vi "run_pharmaBotExp_v0.015.vi"(0 "data in":T12={"daq_ao 1"="Dev1/ao0", "daq_ai 1"="Dev1/ai0", "experiment day folder"=path "C:/multiBot/data/debug/testing", "Multiclamp init error"=0, "Multiclamp Handle Out"=10225184, "sampling rate (Hz)"=20000, "trial name"="t1"}, 1 "auto run?":bool=TRUE, 3 "which manipulator":T13(ring), 4 "HEK/slice options":enum16{"slice", "HEK"}(ring), 5 "error in":errorcluster, 6 "Validate after Experiment":bool, 7 "common cluster":T9, 11 "individual controls in":T8, 13 "images":T3={"slice image"="remote image 000000001461186C", "pipette template"="remote image 000000001461152C", "found pipette"=refnum, "pipette mask for cell tracker"=refnum, "cell images ref"=refnum}) -> (10 "Cell Looks Good?":bool=TRUE, 12 "ValidationOutputCluster":T5(array[cluster]), 14 "ValidationResults":waveform(dbl)[][](array[waveform]), 15 "ValidationPos1":T6(array[ring]), 16 "Exp. Terminated":bool, 17 "ValidationPos2":T6(array[ring]), 18 "ValidationWaveform":waveform(dbl)[](array[waveform]), 19 "error out":errorcluster)   [LabVIEW 2015] (continued)
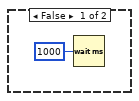
[diagram p2: hidden frame]
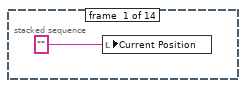
[diagram p3: hidden frame]
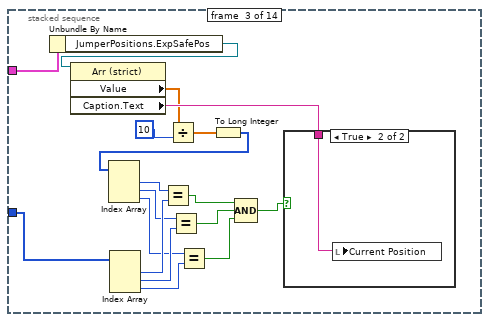
[diagram p5: hidden frame]
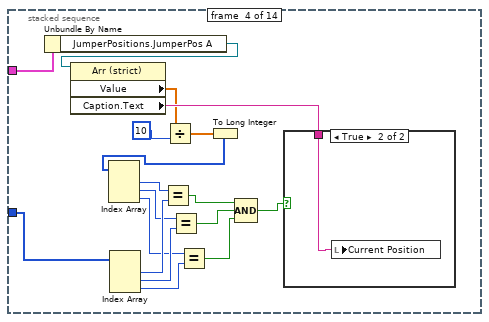
[diagram p7: hidden frame]
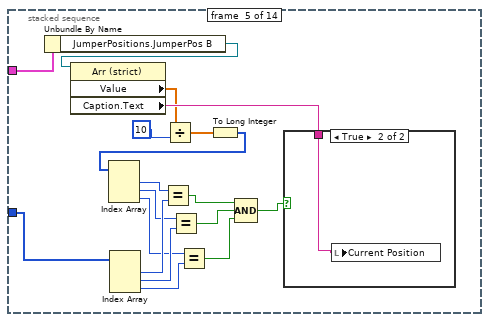
[diagram p9: hidden frame]
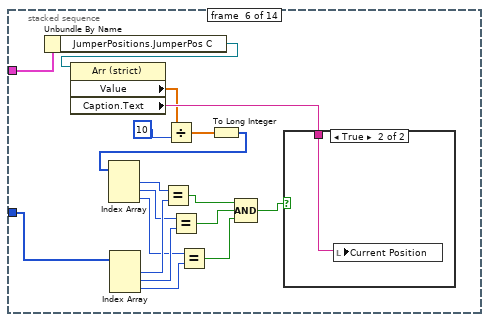
[diagram p11: hidden frame]
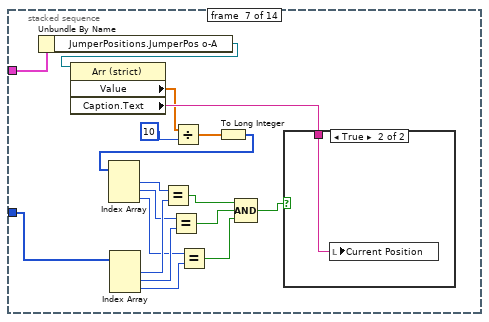
[diagram p13: hidden frame]
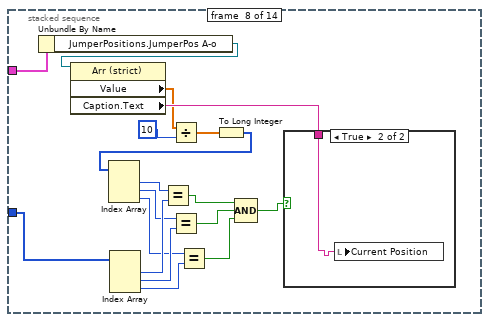
[diagram p15: hidden frame]
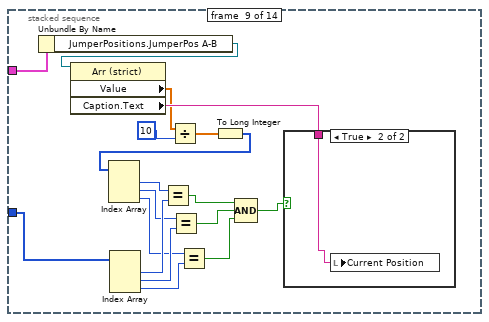
[diagram p17: hidden frame]
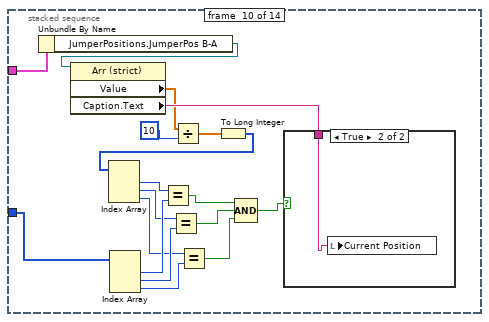
[diagram p19: hidden frame]
            n2141 = control-ref of="PhaseC Experiment Option"() -> (w2881:refnum<vi>)
            n2142 = control-ref of="PhaseE Experiment Option"() -> (w2873:refnum<vi>)
            n2143 = property class="CmbBox"(reference=w2892, "Visible"=TRUE) -> ()  [unwired: 1 in, 2 out]
            n2144 = property class="CmbBox"(reference=w2890, "Visible"=TRUE) -> ()  [unwired: 1 in, 2 out]
            n2145 = property class="CmbBox"(reference=w2872, "Visible"=TRUE) -> ()  [unwired: 1 in, 2 out]
            n2146 = property class="CmbBox"(reference=w2880, "Visible"=TRUE) -> ()  [unwired: 1 in, 2 out]
            n2147 = property class="CmbBox"(reference=w2881, "Visible"=TRUE) -> ()  [unwired: 1 in, 2 out]
            n2148 = property class="CmbBox"(reference=w2873, "Visible"=TRUE) -> ()  [unwired: 1 in, 2 out]
            n2149 = control-ref of="Experiment Selection B"() -> (w2887:refnum<vi>)
            n2150 = control-ref of="Experiment Selection F"() -> (w2869:refnum<vi>)
            n2151 = control-ref of="Experiment Selection D"() -> (w2877:refnum<vi>)
            n2152 = control-ref of="Experiment Selection A"() -> (w2885:refnum<vi>)
            n2153 = control-ref of="Experiment Selection C"() -> (w2884:refnum<vi>)
            n2154 = control-ref of="Experiment Selection E"() -> (w2876:refnum<vi>)
            n2155 = property class="TabCtl (strict)"(reference=w2887, "Visible"=TRUE) -> ()  [unwired: 1 in, 2 out]
            n2156 = property class="TabCtl (strict)"(reference=w2885, "Visible"=TRUE) -> ()  [unwired: 1 in, 2 out]
            n2157 = property class="TabCtl (strict)"(reference=w2869, "Visible"=TRUE) -> ()  [unwired: 1 in, 2 out]
            n2158 = property class="TabCtl (strict)"(reference=w2877, "Visible"=TRUE) -> ()  [unwired: 1 in, 2 out]
            n2159 = property class="TabCtl (strict)"(reference=w2884, "Visible"=TRUE) -> ()  [unwired: 1 in, 2 out]
            n2160 = property class="TabCtl (strict)"(reference=w2876, "Visible"=TRUE) -> ()  [unwired: 1 in, 2 out]
            n2161 = control-ref of="PhaseH Experiment Option"() -> (w2847:refnum<vi>)
            n2162 = control-ref of="PhaseL Experiment Option"() -> (w2865:refnum<vi>)
            n2163 = control-ref of="PhaseG Experiment Option"() -> (w2845:refnum<vi>)
            n2164 = control-ref of="PhaseJ Experiment Option"() -> (w2857:refnum<vi>)
            n2165 = control-ref of="PhaseI Experiment Option"() -> (w2856:refnum<vi>)
            n2166 = control-ref of="PhaseK Experiment Option"() -> (w2864:refnum<vi>)
            n2167 = property class="CmbBox"(reference=w2845, "Visible"=TRUE) -> ()  [unwired: 1 in, 2 out]
            n2168 = property class="CmbBox"(reference=w2847, "Visible"=TRUE) -> ()  [unwired: 1 in, 2 out]
            n2169 = property class="CmbBox"(reference=w2865, "Visible"=FALSE) -> ()  [unwired: 1 in, 2 out]
            n2170 = property class="CmbBox"(reference=w2857, "Visible"=TRUE) -> ()  [unwired: 1 in, 2 out]
            n2171 = property class="CmbBox"(reference=w2856, "Visible"=TRUE) -> ()  [unwired: 1 in, 2 out]
            n2172 = property class="CmbBox"(reference=w2864, "Visible"=FALSE) -> ()  [unwired: 1 in, 2 out]
            n2173 = control-ref of="Experiment Selection H"() -> (w2850:refnum<vi>)
            n2174 = control-ref of="Experiment Selection L"() -> (w2868:refnum<vi>)
            n2175 = control-ref of="Experiment Selection J"() -> (w2860:refnum<vi>)
            n2176 = control-ref of="Experiment Selection G"() -> (w2852:refnum<vi>)
            n2177 = control-ref of="Experiment Selection I"() -> (w2853:refnum<vi>)
            n2178 = control-ref of="Experiment Selection K"() -> (w2861:refnum<vi>)
            n2179 = property class="TabCtl (strict)"(reference=w2850, "Visible"=TRUE) -> ()  [unwired: 1 in, 2 out]
            n2180 = property class="TabCtl (strict)"(reference=w2852, "Visible"=TRUE) -> ()  [unwired: 1 in, 2 out]
            n2181 = property class="TabCtl (strict)"(reference=w2868, "Visible"=FALSE) -> ()  [unwired: 1 in, 2 out]
            n2182 = property class="TabCtl (strict)"(reference=w2860, "Visible"=TRUE) -> ()  [unwired: 1 in, 2 out]
            n2183 = property class="TabCtl (strict)"(reference=w2853, "Visible"=TRUE) -> ()  [unwired: 1 in, 2 out]
            n2184 = property class="TabCtl (strict)"(reference=w2861, "Visible"=FALSE) -> ()  [unwired: 1 in, 2 out]
          }
          frame 11 {
            n2185 = control-ref of="PhaseB Experiment Option"() -> (w2938:refnum<vi>)
            n2186 = control-ref of="PhaseF Experiment Option"() -> (w2920:refnum<vi>)
            n2187 = control-ref of="PhaseA Experiment Option"() -> (w2940:refnum<vi>)
            n2188 = control-ref of="PhaseD Experiment Option"() -> (w2928:refnum<vi>)
            n2189 = control-ref of="PhaseC Experiment Option"() -> (w2929:refnum<vi>)
            n2190 = control-ref of="PhaseE Experiment Option"() -> (w2921:refnum<vi>)
            n2191 = property class="CmbBox"(reference=w2940, "Visible"=TRUE) -> ()  [unwired: 1 in, 2 out]
            n2192 = property class="CmbBox"(reference=w2938, "Visible"=TRUE) -> ()  [unwired: 1 in, 2 out]
            n2193 = property class="CmbBox"(reference=w2920, "Visible"=TRUE) -> ()  [unwired: 1 in, 2 out]
            n2194 = property class="CmbBox"(reference=w2928, "Visible"=TRUE) -> ()  [unwired: 1 in, 2 out]
            n2195 = property class="CmbBox"(reference=w2929, "Visible"=TRUE) -> ()  [unwired: 1 in, 2 out]
            n2196 = property class="CmbBox"(reference=w2921, "Visible"=TRUE) -> ()  [unwired: 1 in, 2 out]
            n2197 = control-ref of="Experiment Selection B"() -> (w2935:refnum<vi>)
            n2198 = control-ref of="Experiment Selection F"() -> (w2917:refnum<vi>)
            n2199 = control-ref of="Experiment Selection D"() -> (w2925:refnum<vi>)
            n2200 = control-ref of="Experiment Selection A"() -> (w2933:refnum<vi>)
            n2201 = control-ref of="Experiment Selection C"() -> (w2932:refnum<vi>)
            n2202 = control-ref of="Experiment Selection E"() -> (w2924:refnum<vi>)
            n2203 = property class="TabCtl (strict)"(reference=w2935, "Visible"=TRUE) -> ()  [unwired: 1 in, 2 out]
            n2204 = property class="TabCtl (strict)"(reference=w2933, "Visible"=TRUE) -> ()  [unwired: 1 in, 2 out]
            n2205 = property class="TabCtl (strict)"(reference=w2917, "Visible"=TRUE) -> ()  [unwired: 1 in, 2 out]
            n2206 = property class="TabCtl (strict)"(reference=w2925, "Visible"=TRUE) -> ()  [unwired: 1 in, 2 out]
            n2207 = property class="TabCtl (strict)"(reference=w2932, "Visible"=TRUE) -> ()  [unwired: 1 in, 2 out]
            n2208 = property class="TabCtl (strict)"(reference=w2924, "Visible"=TRUE) -> ()  [unwired: 1 in, 2 out]
            n2209 = control-ref of="PhaseH Experiment Option"() -> (w2895:refnum<vi>)
            n2210 = control-ref of="PhaseL Experiment Option"() -> (w2913:refnum<vi>)
            n2211 = control-ref of="PhaseG Experiment Option"() -> (w2893:refnum<vi>)
            n2212 = control-ref of="PhaseJ Experiment Option"() -> (w2905:refnum<vi>)
            n2213 = control-ref of="PhaseI Experiment Option"() -> (w2904:refnum<vi>)
            n2214 = control-ref of="PhaseK Experiment Option"() -> (w2912:refnum<vi>)
            n2215 = property class="CmbBox"(reference=w2893, "Visible"=TRUE) -> ()  [unwired: 1 in, 2 out]
            n2216 = property class="CmbBox"(reference=w2895, "Visible"=TRUE) -> ()  [unwired: 1 in, 2 out]
            n2217 = property class="CmbBox"(reference=w2913, "Visible"=FALSE) -> ()  [unwired: 1 in, 2 out]
            n2218 = property class="CmbBox"(reference=w2905, "Visible"=TRUE) -> ()  [unwired: 1 in, 2 out]
            n2219 = property class="CmbBox"(reference=w2904, "Visible"=TRUE) -> ()  [unwired: 1 in, 2 out]
            n2220 = property class="CmbBox"(reference=w2912, "Visible"=TRUE) -> ()  [unwired: 1 in, 2 out]
            n2221 = control-ref of="Experiment Selection H"() -> (w2898:refnum<vi>)
            n2222 = control-ref of="Experiment Selection L"() -> (w2916:refnum<vi>)
            n2223 = control-ref of="Experiment Selection J"() -> (w2908:refnum<vi>)
            n2224 = control-ref of="Experiment Selection G"() -> (w2900:refnum<vi>)
            n2225 = control-ref of="Experiment Selection I"() -> (w2901:refnum<vi>)
            n2226 = control-ref of="Experiment Selection K"() -> (w2909:refnum<vi>)
            n2227 = property class="TabCtl (strict)"(reference=w2898, "Visible"=TRUE) -> ()  [unwired: 1 in, 2 out]
            n2228 = property class="TabCtl (strict)"(reference=w2900, "Visible"=TRUE) -> ()  [unwired: 1 in, 2 out]
            n2229 = property class="TabCtl (strict)"(reference=w2916, "Visible"=FALSE) -> ()  [unwired: 1 in, 2 out]
            n2230 = property class="TabCtl (strict)"(reference=w2908, "Visible"=TRUE) -> ()  [unwired: 1 in, 2 out]
            n2231 = property class="TabCtl (strict)"(reference=w2901, "Visible"=TRUE) -> ()  [unwired: 1 in, 2 out]
            n2232 = property class="TabCtl (strict)"(reference=w2909, "Visible"=TRUE) -> ()  [unwired: 1 in, 2 out]
          }
          frame 12 {
            n2233 = control-ref of="PhaseB Experiment Option"() -> (w2986:refnum<vi>)
            n2234 = control-ref of="PhaseF Experiment Option"() -> (w2968:refnum<vi>)
            n2235 = control-ref of="PhaseA Experiment Option"() -> (w2988:refnum<vi>)
            n2236 = control-ref of="PhaseD Experiment Option"() -> (w2976:refnum<vi>)
            n2237 = control-ref of="PhaseC Experiment Option"() -> (w2977:refnum<vi>)
            n2238 = control-ref of="PhaseE Experiment Option"() -> (w2969:refnum<vi>)
            n2239 = property class="CmbBox"(reference=w2988, "Visible"=TRUE) -> ()  [unwired: 1 in, 2 out]
            n2240 = property class="CmbBox"(reference=w2986, "Visible"=TRUE) -> ()  [unwired: 1 in, 2 out]
            n2241 = property class="CmbBox"(reference=w2968, "Visible"=TRUE) -> ()  [unwired: 1 in, 2 out]
            n2242 = property class="CmbBox"(reference=w2976, "Visible"=TRUE) -> ()  [unwired: 1 in, 2 out]
            n2243 = property class="CmbBox"(reference=w2977, "Visible"=TRUE) -> ()  [unwired: 1 in, 2 out]
            n2244 = property class="CmbBox"(reference=w2969, "Visible"=TRUE) -> ()  [unwired: 1 in, 2 out]
            n2245 = control-ref of="Experiment Selection B"() -> (w2983:refnum<vi>)
            n2246 = control-ref of="Experiment Selection F"() -> (w2965:refnum<vi>)
            n2247 = control-ref of="Experiment Selection D"() -> (w2973:refnum<vi>)
            n2248 = control-ref of="Experiment Selection A"() -> (w2981:refnum<vi>)
            n2249 = control-ref of="Experiment Selection C"() -> (w2980:refnum<vi>)
            n2250 = control-ref of="Experiment Selection E"() -> (w2972:refnum<vi>)
            n2251 = property class="TabCtl (strict)"(reference=w2983, "Visible"=TRUE) -> ()  [unwired: 1 in, 2 out]
            n2252 = property class="TabCtl (strict)"(reference=w2981, "Visible"=TRUE) -> ()  [unwired: 1 in, 2 out]
            n2253 = property class="TabCtl (strict)"(reference=w2965, "Visible"=TRUE) -> ()  [unwired: 1 in, 2 out]
            n2254 = property class="TabCtl (strict)"(reference=w2973, "Visible"=TRUE) -> ()  [unwired: 1 in, 2 out]
            n2255 = property class="TabCtl (strict)"(reference=w2980, "Visible"=TRUE) -> ()  [unwired: 1 in, 2 out]
            n2256 = property class="TabCtl (strict)"(reference=w2972, "Visible"=TRUE) -> ()  [unwired: 1 in, 2 out]
            n2257 = control-ref of="PhaseH Experiment Option"() -> (w2943:refnum<vi>)
            n2258 = control-ref of="PhaseL Experiment Option"() -> (w2961:refnum<vi>)
            n2259 = control-ref of="PhaseG Experiment Option"() -> (w2941:refnum<vi>)
            n2260 = control-ref of="PhaseJ Experiment Option"() -> (w2953:refnum<vi>)
            n2261 = control-ref of="PhaseI Experiment Option"() -> (w2952:refnum<vi>)
            n2262 = control-ref of="PhaseK Experiment Option"() -> (w2960:refnum<vi>)
            n2263 = property class="CmbBox"(reference=w2941, "Visible"=TRUE) -> ()  [unwired: 1 in, 2 out]
            n2264 = property class="CmbBox"(reference=w2943, "Visible"=TRUE) -> ()  [unwired: 1 in, 2 out]
            n2265 = property class="CmbBox"(reference=w2961, "Visible"=TRUE) -> ()  [unwired: 1 in, 2 out]
            n2266 = property class="CmbBox"(reference=w2953, "Visible"=TRUE) -> ()  [unwired: 1 in, 2 out]
            n2267 = property class="CmbBox"(reference=w2952, "Visible"=TRUE) -> ()  [unwired: 1 in, 2 out]
            n2268 = property class="CmbBox"(reference=w2960, "Visible"=TRUE) -> ()  [unwired: 1 in, 2 out]
            n2269 = control-ref of="Experiment Selection H"() -> (w2946:refnum<vi>)
            n2270 = control-ref of="Experiment Selection L"() -> (w2964:refnum<vi>)
            n2271 = control-ref of="Experiment Selection J"() -> (w2956:refnum<vi>)
            n2272 = control-ref of="Experiment Selection G"() -> (w2948:refnum<vi>)
            n2273 = control-ref of="Experiment Selection I"() -> (w2949:refnum<vi>)
            n2274 = control-ref of="Experiment Selection K"() -> (w2957:refnum<vi>)
            n2275 = property class="TabCtl (strict)"(reference=w2946, "Visible"=TRUE) -> ()  [unwired: 1 in, 2 out]
            n2276 = property class="TabCtl (strict)"(reference=w2948, "Visible"=TRUE) -> ()  [unwired: 1 in, 2 out]
            n2277 = property class="TabCtl (strict)"(reference=w2964, "Visible"=TRUE) -> ()  [unwired: 1 in, 2 out]
            n2278 = property class="TabCtl (strict)"(reference=w2956, "Visible"=TRUE) -> ()  [unwired: 1 in, 2 out]
            n2279 = property class="TabCtl (strict)"(reference=w2949, "Visible"=TRUE) -> ()  [unwired: 1 in, 2 out]
            n2280 = property class="TabCtl (strict)"(reference=w2957, "Visible"=TRUE) -> ()  [unwired: 1 in, 2 out]
          }
        }
      }
      event "Single Manip Jump A", "Single Manip Jump B", "Single Manip Jump C", "Single Manip Jump D", "Single Manip Jump E", "Single Manip Jump F", "Single Manip Jump L", "Single Manip Jump K", "Single Manip Jump J", "Single Manip Jump I", "Single Manip Jump H", "Single Manip Jump G": Value Change {
        n2281 = event-data() -> ("CtlRef"=w2992:refnum<vi>, "OldVal"=w2990:T28, "NewVal"=w2991:T28)  [unwired: 1 in, 3 out]
        n2282 = local read "Waveform Simulation sampling rate (Hz)"() -> (w2989:i32)
        n2283 = call "calc_singleManipJumpWaveform_v0.02.vi"("New input cluster"=w2991, "Old input cluster"=w2990, "simulate Wave freq"=w2989) -> ("output cluster"=w2993:T28)  [unwired: 11 in, 1 out]
        n2284 = property class="Clust (strict)"(reference=w2992, "Value"=w2993) -> ()  [unwired: 1 in, 2 out]
      }
      event "Multi Manip Jump A", "Multi Manip Jump B", "Multi Manip Jump C", "Multi Manip Jump D", "Multi Manip Jump E", "Multi Manip Jump F", "Multi Manip Jump L", "Multi Manip Jump K", "Multi Manip Jump J", "Multi Manip Jump I", "Multi Manip Jump H", "Multi Manip Jump G": Value Change {
        n2285 = event-data() -> ("CtlRef"=w2997:refnum<vi>, "OldVal"=w2995:T30, "NewVal"=w2996:T30)  [unwired: 1 in, 3 out]
        n2286 = local read "Waveform Simulation sampling rate (Hz)"() -> (w2994:i32)
        n2287 = call "calc_multiManipJumpWaveform_v0.02.vi"("New input cluster"=w2996, "Old input cluster"=w2995, "Numeric"=w2994) -> ("output cluster"=w2998:T30)  [unwired: 11 in, 1 out]
        n2288 = property class="Clust (strict)"(reference=w2997, "Value"=w2998) -> ()  [unwired: 1 in, 2 out]
      }
      event "Paired Pulse A", "Paired Pulse B", "Paired Pulse C", "Paired Pulse D", "Paired Pulse E", "Paired Pulse F", "Paired Pulse L", "Paired Pulse K", "Paired Pulse J", "Paired Pulse I", "Paired Pulse H", "Paired Pulse G": Value Change {
        n2289 = event-data() -> ("CtlRef"=w3003:refnum<vi>, "OldVal"=w3001:T27, "NewVal"=w3002:T27)  [unwired: 1 in, 3 out]
        n2290 = local read "Waveform Simulation Jump Filter (Hz)"() -> (w3000:dbl)
        n2291 = local read "Waveform Simulation sampling rate (Hz)"() -> (w2999:i32)
        n2292 = call "calc_PairedPulseWaveform_v0.02.vi"("New input cluster"=w3002, "Old input cluster"=w3001, "Numeric"=w2999, "Jump Filter Freq (Hz)"=w3000) -> ("output cluster"=w3004:T27)  [unwired: 10 in, 1 out]
        n2293 = property class="Clust (strict)"(reference=w3003, "Value"=w3004) -> ()  [unwired: 1 in, 2 out]
      }
      event "Jump Train A", "Jump Train B", "Jump Train C", "Jump Train D", "Jump Train E", "Jump Train F", "Jump Train L", "Jump Train K", "Jump Train J", "Jump Train I", "Jump Train H", "Jump Train G": Value Change {
        n2294 = event-data() -> ("CtlRef"=w3009:refnum<vi>, "OldVal"=w3007:T26, "NewVal"=w3008:T26)  [unwired: 1 in, 3 out]
        n2295 = local read "Waveform Simulation Jump Filter (Hz)"() -> (w3006:dbl)
        n2296 = local read "Waveform Simulation sampling rate (Hz)"() -> (w3005:i32)
        n2297 = call "calc_jumpTrainWaveform_v0.03.vi"("New input cluster"=w3008, "Old input cluster"=w3007, "sample freq"=w3005, "Jump Filter Freq (Hz)"=w3006) -> ("output cluster"=w3010:T26)  [unwired: 10 in, 1 out]
        n2298 = property class="Clust (strict)"(reference=w3009, "Value"=w3010) -> ()  [unwired: 1 in, 2 out]
      }
      event "Single Jump A", "Single Jump B", "Single Jump C", "Single Jump D", "Single Jump E", "Single Jump F", "Single Jump L", "Single Jump K", "Single Jump J", "Single Jump I", "Single Jump H", "Single Jump G": Value Change {
        n2299 = event-data() -> ("CtlRef"=w3015:refnum<vi>, "OldVal"=w3013:T21, "NewVal"=w3014:T21)  [unwired: 1 in, 3 out]
        n2300 = local read "Waveform Simulation Jump Filter (Hz)"() -> (w3012:dbl)
        n2301 = local read "Waveform Simulation sampling rate (Hz)"() -> (w3011:i32)
        n2302 = call "calc_sinlge JumpWaveform_v0.03.vi"("New input cluster"=w3014, "Old input cluster"=w3013, "sample freq"=w3011, "Jump Filter Freq (Hz)"=w3012) -> ("output cluster"=w3016:T21)  [unwired: 10 in, 1 out]
        n2303 = property class="Clust (strict)"(reference=w3015, "Value"=w3016) -> ()  [unwired: 1 in, 2 out]
      }
      event "Solution Change A", "Solution Change B", "Solution Change C", "Solution Change D", "Solution Change E", "Solution Change F", "Solution Change L", "Solution Change K", "Solution Change J", "Solution Change I", "Solution Change H", "Solution Change G": Value Change {
        n2304 = event-data() -> ("CtlRef"=w3020:refnum<vi>, "OldVal"=w3018:T22, "NewVal"=w3019:T22)  [unwired: 1 in, 3 out]
        n2305 = local read "Waveform Simulation sampling rate (Hz)"() -> (w3017:i32)
        n2306 = call "calc_SolutionChangeWaveform_v0.03.vi"("New input cluster"=w3019, "Old input cluster"=w3018, "sample freq"=w3017) -> ("output cluster"=w3021:T22)  [unwired: 11 in, 1 out]
        n2307 = property class="Clust (strict)"(reference=w3020, "Value"=w3021) -> ()  [unwired: 1 in, 2 out]
      }
      event "Voltage Ramp A", "Voltage Ramp B", "Voltage Ramp C", "Voltage Ramp D", "Voltage Ramp E", "Voltage Ramp F", "Voltage Ramp L", "Voltage Ramp K", "Voltage Ramp J", "Voltage Ramp I", "Voltage Ramp H", "Voltage Ramp G": Value Change {
        n2308 = event-data() -> ("CtlRef"=w3025:refnum<vi>, "OldVal"=w3023:T24, "NewVal"=w3024:T24)  [unwired: 1 in, 3 out]
        n2309 = local read "Waveform Simulation sampling rate (Hz)"() -> (w3022:i32)
        n2310 = call "calc_VoltageRampWaveform_v0.03.vi"("New input cluster"=w3024, "Old input cluster"=w3023, "sample freq"=w3022) -> ("output cluster"=w3026:T24)  [unwired: 11 in, 1 out]
        n2311 = property class="Clust (strict)"(reference=w3025, "Value"=w3026) -> ()  [unwired: 1 in, 2 out]
      }
      event "Current Ramp A", "Current Ramp B", "Current Ramp C", "Current Ramp D", "Current Ramp E", "Current Ramp F", "Current Ramp G", "Current Ramp H", "Current Ramp I", "Current Ramp J", "Current Ramp K", "Current Ramp L": Value Change {
        n2312 = event-data() -> ("CtlRef"=w3030:refnum<vi>, "OldVal"=w3028:T32, "NewVal"=w3029:T32)  [unwired: 1 in, 3 out]
        n2313 = local read "Waveform Simulation sampling rate (Hz)"() -> (w3027:i32)
        n2314 = call "calc_CurrentRampWaveform_v0.03.vi"("New input cluster"=w3029, "Old input cluster"=w3028, "sample freq"=w3027) -> ("output cluster"=w3031:T32)  [unwired: 11 in, 1 out]
        n2315 = property class="Clust (strict)"(reference=w3030, "Value"=w3031) -> ()  [unwired: 1 in, 2 out]
      }
      event "Voltage Step A", "Voltage Step B", "Voltage Step C", "Voltage Step D", "Voltage Step E", "Voltage Step F", "Voltage Step L", "Voltage Step K", "Voltage Step J", "Voltage Step I", "Voltage Step H", "Voltage Step G": Value Change {
        n2316 = event-data() -> ("CtlRef"=w3035:refnum<vi>, "OldVal"=w3033:T23, "NewVal"=w3034:T23)  [unwired: 1 in, 3 out]
        n2317 = local read "Waveform Simulation sampling rate (Hz)"() -> (w3032:i32)
        n2318 = call "calc_VoltageStepWaveform_v0.03.vi"("New input cluster"=w3034, "Old input cluster"=w3033, "sample freq"=w3032) -> ("output cluster"=w3036:T23)  [unwired: 11 in, 1 out]
        n2319 = property class="Clust (strict)"(reference=w3035, "Value"=w3036) -> ()  [unwired: 1 in, 2 out]
      }
      event "Voltage Pulse A", "Voltage Pulse B", "Voltage Pulse C", "Voltage Pulse D", "Voltage Pulse E", "Voltage Pulse F", "Voltage Pulse L", "Voltage Pulse K", "Voltage Pulse J", "Voltage Pulse I", "Voltage Pulse H", "Voltage Pulse G": Value Change {
        n2320 = event-data() -> ("CtlRef"=w3040:refnum<vi>, "OldVal"=w3038:T25, "NewVal"=w3039:T25)  [unwired: 1 in, 3 out]
        n2321 = local read "Waveform Simulation sampling rate (Hz)"() -> (w3037:i32)
        n2322 = call "calc_VoltagepulseWaveform_v0.03.vi"("New input cluster"=w3039, "Old input cluster"=w3038, "sample freq"=w3037) -> ("output cluster"=w3041:T25)  [unwired: 11 in, 1 out]
        n2323 = property class="Clust (strict)"(reference=w3040, "Value"=w3041) -> ()  [unwired: 1 in, 2 out]
      }
      event "Current Pulse A", "Current Pulse B", "Current Pulse C", "Current Pulse D", "Current Pulse E", "Current Pulse F", "Current Pulse G", "Current Pulse H", "Current Pulse I", "Current Pulse J", "Current Pulse K", "Current Pulse L": Value Change {
        n2324 = event-data() -> ("CtlRef"=w3045:refnum<vi>, "OldVal"=w3043:T31, "NewVal"=w3044:T31)  [unwired: 1 in, 3 out]
        n2325 = local read "Waveform Simulation sampling rate (Hz)"() -> (w3042:i32)
        n2326 = call "calc_CurrentpulseWaveform_v0.03.vi"("New input cluster"=w3044, "Old input cluster"=w3043, "sample freq"=w3042) -> ("output cluster"=w3046:T31)  [unwired: 11 in, 1 out]
        n2327 = property class="Clust (strict)"(reference=w3045, "Value"=w3046) -> ()  [unwired: 1 in, 2 out]
      }
      event "update plots": Value Change {
        n2328 = event-data() -> ("NewVal"=w3054:bool)  [unwired: 1 in, 5 out]
        n2329 = local read "Waveform Simulation Jump Filter (Hz)"() -> (w3048:dbl)
        n2330 = local read "Waveform Simulation sampling rate (Hz)"() -> (w3049:i32)
        n2331 = local read "How Many Experimental Phases?"() -> (w3047:i32)
        n2332 = local read "data in"() -> (w3053:T12)
        n2333 = Unbundle By Name(w3053) -> ("sampling rate (Hz)"=w3052:i32)
        n2334 = case shown="True" w3054 {
          tunnel: w3052 -> [_ w3056]
          tunnel: [FALSE w3061] -> w3051
          tunnel: w3050 -> [_ w3060]
          tunnel: w3048 -> [_ w3059]
          tunnel: w3049 -> [_ w3058]
          tunnel: w3047 -> [_ w3057]
          frame False {
          }
          frame True {
            n2335 = stacked-sequence {
              tunnel: [_ _ _ _ _ _ _ w3097] -> w3061
              tunnel: w3060 -> [_ w3073 _ _ _ _ _ _]
              tunnel: w3059 -> [_ w3072 _ _ _ _ _ _]
              tunnel: w3058 -> [_ w3070 _ _ _ _ _ _]
              tunnel: w3057 -> [_ w3069 _ _ _ _ _ _]
              tunnel: w3056 -> [w3062 _ w3074 _ _ _ _ _]
              frame #0 {
                # "repMemTest Iprot"
                n2336 = local read "repMemTest Iprot"() -> (w3067:T15)
                n2337 = Unbundle By Name(w3067) -> ("Iclamp in"=w3066:T14, "# iter"=w3065:i32, "# reps IC"=w3064:i32)
                n2338 = call "clamp_protocol.vi"("which clamp"=enum16{"VClamp", "IClamp"}."IClamp", "# reps"=w3064, "# Iterations"=w3065, "clamp in"=w3066, "sampling rate (Hz)"=w3062) -> ("View profile (wvfrms)"=→"repMemTest iprot cmd":waveform(dbl)[])  [unwired: 2 out]
              }
              frame #1 {
                n2339 = call "clearOrCalcAllPhaseWaveforms_v02.vi"("How Many Experimental Phases?"=w3069, "Clear Waveform?"=FALSE, "Waveform Simulation Jump Filter (Hz)"=w3072, "Waveform Simulation sampling rate (Hz)"=w3070, "ExperimentOptionsCluster"=w3073) -> ()  [unwired: 6 in, 1 out]
              }
              frame #2 {
                # "repMemTest Vprot"
                n2340 = local read "repMemTest Vprot"() -> (w3078:T16)
                n2341 = Unbundle By Name(w3078) -> ("Vclamp in"=w3079:T14, "# iter"=w3076:i32, "# reps VC"=w3075:i32)
                n2342 = call "clamp_protocol.vi"("which clamp"=enum16{"VClamp", "IClamp"}."VClamp", "# reps"=w3075, "# Iterations"=w3076, "clamp in"=w3079, "sampling rate (Hz)"=w3074) -> ("View profile (wvfrms)"=→"repMemTest vprot cmd":waveform(dbl)[])  [unwired: 2 out]
              }
              frame #3 {
                # "repMemTest Imem"
                n2343 = local read "repMemTest Iclamp memtest"() -> (w3081:T17)
                n2344 = call "ext_cmd_sensitivity.vi"("which clamp"=enum16{"VClamp", "IClamp"}."IClamp") -> ("division factor"=w3084:dbl)  [unwired: 10 in]
                n2345 = call "generate_memtest_pulse.vi"("external cmd sensitivity"=w3084, "memtest"=w3081) -> ("view memtest"=→"repMemTest imemtest view":waveform(dbl))  [unwired: 8 in, 1 out]
              }
              frame #4 {
                # "repMemTest Vmem"
                n2346 = local read "repMemTest Vclamp memtest"() -> (w3085:T17)
                n2347 = call "ext_cmd_sensitivity.vi"("which clamp"=enum16{"VClamp", "IClamp"}."VClamp") -> ("division factor"=w3088:dbl)  [unwired: 10 in]
                n2348 = call "generate_memtest_pulse.vi"("external cmd sensitivity"=w3088, "memtest"=w3085) -> ("view memtest"=→"repMemTest vmemtest view":waveform(dbl))  [unwired: 8 in, 1 out]
              }
              frame #5 {
                # "Holding Imem"
                n2349 = local read "holding Iclamp memtest"() -> (w3089:T17)
                n2350 = call "ext_cmd_sensitivity.vi"("which clamp"=enum16{"VClamp", "IClamp"}."IClamp") -> ("division factor"=w3092:dbl)  [unwired: 10 in]
                n2351 = call "generate_memtest_pulse.vi"("external cmd sensitivity"=w3092, "memtest"=w3089) -> ("view memtest"=→"holding imemtest cmd":waveform(dbl))  [unwired: 8 in, 1 out]
              }
              frame #6 {
                # "Holding Vmem"
                n2352 = local read "holding Vclamp memtest"() -> (w3093:T17)
                n2353 = call "ext_cmd_sensitivity.vi"("which clamp"=enum16{"VClamp", "IClamp"}."VClamp") -> ("division factor"=w3096:dbl)  [unwired: 10 in]
                n2354 = call "generate_memtest_pulse.vi"("external cmd sensitivity"=w3096, "memtest"=w3093) -> ("view memtest"=→"holding vmemtest cmd":waveform(dbl))  [unwired: 8 in, 1 out]
              }
              frame #7 {
                n2355 = local read "auto run?"() -> (w3098:bool)
                n2356 = case shown="True" w3098 {
                  tunnel: [FALSE TRUE] -> w3097
                  frame False {
                  }
                  frame True {
                    n2357 = local write "auto WC run trigger"(TRUE ("auto WC run trigger")) -> ()
                    n2358 = property on="update plots" class="Bool (strict)"("Value"=FALSE ("Value (Signaling)")) -> ()  [unwired: 2 in, 2 out]
                  }
                }
              }
            }
          }
        }
      }
      event "run": Value Change {
        n2359 = event-data() -> ("NewVal"=w3104:bool)  [unwired: 1 in, 5 out]
        n2360 = case shown="True" w3104 {
          selector: w3104 -> [_ w3105]
          frame False {
          }
          frame True {
            n2361 = property on="auto WC run trigger" class="Bool (strict)"("Value"=w3105) -> ()  [unwired: 2 in, 2 out]
          }
        }
      }
      event "Clear Waveforms": Value Change {
        n2362 = event-data() -> ("CtlRef"=w3110:refnum<vi>, "NewVal"=w3111:bool)  [unwired: 1 in, 4 out]
        n2363 = local read "Waveform Simulation Jump Filter (Hz)"() -> (w3108:dbl)
        n2364 = local read "Waveform Simulation sampling rate (Hz)"() -> (w3107:i32)
        n2365 = local read "How Many Experimental Phases?"() -> (w3106:i32)
        n2366 = case shown="True" w3111 {
          tunnel: w3110 -> [_ w3117]
          tunnel: w3109 -> [_ w3116]
          tunnel: w3107 -> [_ w3115]
          tunnel: w3108 -> [_ w3114]
          tunnel: w3106 -> [_ w3112]
          frame False {
          }
          frame True {
            n2367 = flat-sequence {
              tunnel: w3117 -> [w3123]
              tunnel: [w3123] -> w3113
              tunnel: w3116 -> [w3122]
              tunnel: w3115 -> [w3120]
              tunnel: w3114 -> [w3119]
              tunnel: w3112 -> [w3118]
              tunnel: w3113 -> [w3127]
              frame #0 {
                n2368 = call "clearOrCalcAllPhaseWaveforms_v02.vi"("How Many Experimental Phases?"=w3118, "Clear Waveform?"=TRUE, "Waveform Simulation Jump Filter (Hz)"=w3119, "Waveform Simulation sampling rate (Hz)"=w3120, "ExperimentOptionsCluster"=w3122) -> ()  [unwired: 6 in, 1 out]
              }
              frame #1 {
                n2369 = property class="Bool (strict)"(reference=w3127, "Value"=FALSE) -> ()  [unwired: 1 in, 2 out]
                n2370 = One Button Dialog(message="Finished Clearing" ("string"), button name ("OK")="click to resume") -> ()  [unwired: 1 out]
              }
            }
          }
        }
      }
      event "Make Waveforms": Value Change {
        n2371 = event-data() -> ("CtlRef"=w3132:refnum<vi>, "NewVal"=w3133:bool)  [unwired: 1 in, 4 out]
        n2372 = local read "Waveform Simulation Jump Filter (Hz)"() -> (w3129:dbl)
        n2373 = local read "Waveform Simulation sampling rate (Hz)"() -> (w3130:i32)
        n2374 = local read "How Many Experimental Phases?"() -> (w3128:i32)
        n2375 = case shown="True" w3133 {
          tunnel: w3132 -> [_ w3139]
          tunnel: w3131 -> [_ w3138]
          tunnel: w3130 -> [_ w3137]
          tunnel: w3129 -> [_ w3136]
          tunnel: w3128 -> [_ w3134]
          frame False {
          }
          frame True {
            n2376 = flat-sequence {
              tunnel: w3139 -> [w3145]
              tunnel: [w3145] -> w3135
              tunnel: w3138 -> [w3144]
              tunnel: w3137 -> [w3142]
              tunnel: w3136 -> [w3141]
              tunnel: w3134 -> [w3140]
              tunnel: w3135 -> [w3149]
              frame #0 {
                n2377 = call "clearOrCalcAllPhaseWaveforms_v02.vi"("How Many Experimental Phases?"=w3140, "Clear Waveform?"=FALSE, "Waveform Simulation Jump Filter (Hz)"=w3141, "Waveform Simulation sampling rate (Hz)"=w3142, "ExperimentOptionsCluster"=w3144) -> ()  [unwired: 6 in, 1 out]
              }
              frame #1 {
                n2378 = property class="Bool (strict)"(reference=w3149, "Value"=FALSE) -> ()  [unwired: 1 in, 2 out]
                n2379 = One Button Dialog(message="Finished Making Waveforms" ("string"), button name ("OK")="click to resume") -> ()  [unwired: 1 out]
              }
            }
          }
        }
      }
      event "save", "save as...": Value Change {
        n2380 = event-data() -> ("CtlRef"=w3156:refnum<vi>, "NewVal"=w3155:bool)  [unwired: 1 in, 4 out]
        n2381 = local read "save as..."() -> (w3150:bool)
        n2382 = local read "Waveform Simulation Jump Filter (Hz)"() -> (w3152:dbl)
        n2383 = local read "Waveform Simulation sampling rate (Hz)"() -> (w3151:i32)
        n2384 = local read "How Many Experimental Phases?"() -> (w3153:i32)
        n2385 = case shown="True" w3155 {
          tunnel: w3150 -> [_ w3171]
          tunnel: w3159 -> [_ w3170]
          tunnel: w3158 -> [_ w3169]
          tunnel: w3156 -> [_ w3168]
          tunnel: w3154 -> [_ w3163]
          tunnel: w3151 -> [_ w3162]
          tunnel: w3152 -> [_ w3161]
          tunnel: w3153 -> [_ w3160]
          frame False {
          }
          frame True {
            n2386 = flat-sequence {
              tunnel: w3168 -> [w3178]
              tunnel: w3169 -> [w3179]
              tunnel: w3170 -> [w3180]
              tunnel: w3171 -> [w3181]
              tunnel: [w3181] -> w3167
              tunnel: [w3180] -> w3166
              tunnel: [w3179] -> w3165
              tunnel: [w3178] -> w3164
              tunnel: w3163 -> [w3177]
              tunnel: w3162 -> [w3175]
              tunnel: w3161 -> [w3174]
              tunnel: w3160 -> [w3173]
              tunnel: [w3184] -> w3172
              tunnel: w3167 -> [w3187]
              tunnel: w3166 -> [w3186]
              tunnel: w3165 -> [w3185]
              tunnel: w3164 -> [w3184]
              tunnel: w3172 -> [w3205]
              tunnel: w3163 -> [w3200]
              tunnel: w3162 -> [w3199]
              tunnel: w3161 -> [w3198]
              tunnel: w3160 -> [w3197]
              frame #0 {
                n2387 = call "clearOrCalcAllPhaseWaveforms_v02.vi"("How Many Experimental Phases?"=w3173, "Clear Waveform?"=TRUE, "Waveform Simulation Jump Filter (Hz)"=w3174, "Waveform Simulation sampling rate (Hz)"=w3175, "ExperimentOptionsCluster"=w3177) -> ()  [unwired: 6 in, 1 out]
              }
              frame #1 {
                n2388 = case shown="True" w3187 {
                  tunnel: w3186 -> [w3193 _]
                  tunnel: [w3193 w3195] -> w3183
                  tunnel: [FALSE ("cancelled") w3194] -> w3182
                  frame False {
                  }
                  frame True {
                    n2389 = call "select config"("prompt"="Save as...") -> ("selected path"=w3195:path, "cancelled"=w3194:bool)  [unwired: 11 in, 2 out]
                    n2390 = local write "config file"(w3195) -> ()
                  }
                }
                n2391 = case shown="False" w3182 {
                  tunnel: w3185 -> [w3189 _]
                  tunnel: w3183 -> [w3190 _]
                  frame False {
                    n2392 = call "condition_control_array_v02.vi"("control array in"=w3189) -> ("control array out"=w3188:refnum<vi>[])  [unwired: 9 in, 1 out]
                    n2393 = call "Read and Write Controls to Automatic Config File.vi"("Action"=RWC_Actions."Write", "Control References"=w3188, "filepath"=w3190) -> ()  [unwired: 8 in, 1 out]
                  }
                  frame True {
                  }
                }
              }
              frame #2 {
                n2394 = property class="Bool (strict)"(reference=w3205, "Value"=FALSE) -> ()  [unwired: 1 in, 2 out]
                n2395 = call "clearOrCalcAllPhaseWaveforms_v02.vi"("How Many Experimental Phases?"=w3197, "Clear Waveform?"=FALSE, "Waveform Simulation Jump Filter (Hz)"=w3198, "Waveform Simulation sampling rate (Hz)"=w3199, "ExperimentOptionsCluster"=w3200) -> ()  [unwired: 6 in, 1 out]
                n2396 = One Button Dialog(message="Finished Saving" ("string"), button name ("OK")="click to resume") -> ()  [unwired: 1 out]
              }
            }
          }
        }
      }
      event "load": Value Change {
        n2397 = event-data() -> ("CtlRef"=w3208:refnum<vi>, "NewVal"=w3207:bool)  [unwired: 1 in, 4 out]
        n2398 = case shown="True" w3207 {
          tunnel: w3209 -> [_ w3245]
          tunnel: w3208 -> [_ w3244]
          tunnel: w3206 -> [_ w3215]
          frame False {
          }
          frame True {
            n2399 = flat-sequence {
              tunnel: [w3252] -> w3249
              tunnel: w3245 -> [w3252]
              tunnel: [w3251] -> w3248
              tunnel: w3244 -> [w3251]
              tunnel: w3249 -> [w3257]
              tunnel: [w3254] -> w3247
              tunnel: w3248 -> [w3254]
              tunnel: [w3253] -> w3242
              tunnel: w3247 -> [w3302]
              tunnel: [w3302] -> w3246
              tunnel: [w3301] -> w3243
              tunnel: w3242 -> [w3301]
              tunnel: [w3300] -> w3241
              tunnel: [w3299] -> w3240
              tunnel: [w3297] -> w3239
              tunnel: [w3296] -> w3238
              tunnel: [w3295] -> w3237
              tunnel: [w3294] -> w3236
              tunnel: [w3293] -> w3235
              tunnel: [w3292] -> w3234
              tunnel: [w3291] -> w3233
              tunnel: [w3290] -> w3232
              tunnel: [w3289] -> w3231
              tunnel: [w3288] -> w3230
              tunnel: [w3287] -> w3229
              tunnel: [w3286] -> w3228
              tunnel: [w3285] -> w3227
              tunnel: [w3284] -> w3226
              tunnel: [w3283] -> w3225
              tunnel: [w3282] -> w3224
              tunnel: [w3281] -> w3223
              tunnel: [w3280] -> w3222
              tunnel: [w3279] -> w3221
              tunnel: [w3278] -> w3220
              tunnel: [w3277] -> w3219
              tunnel: [w3276] -> w3218
              tunnel: [w3275] -> w3217
              tunnel: [w3274] -> w3216
              tunnel: w3246 -> [w3331]
              tunnel: w3243 -> [_]
              tunnel: w3241 -> [w3304]
              tunnel: w3240 -> [w3303]
              tunnel: w3239 -> [w3328]
              tunnel: w3238 -> [w3327]
              tunnel: w3237 -> [w3326]
              tunnel: w3236 -> [w3325]
              tunnel: w3235 -> [w3324]
              tunnel: w3234 -> [w3323]
              tunnel: w3233 -> [w3322]
              tunnel: w3232 -> [w3321]
              tunnel: w3231 -> [w3320]
              tunnel: w3230 -> [w3319]
              tunnel: w3229 -> [w3318]
              tunnel: w3228 -> [w3317]
              tunnel: w3227 -> [w3316]
              tunnel: w3226 -> [w3315]
              tunnel: w3225 -> [w3314]
              tunnel: w3224 -> [w3313]
              tunnel: w3223 -> [w3312]
              tunnel: w3222 -> [w3311]
              tunnel: w3221 -> [w3310]
              tunnel: w3220 -> [w3309]
              tunnel: w3219 -> [w3308]
              tunnel: w3218 -> [w3307]
              tunnel: w3217 -> [w3306]
              tunnel: w3216 -> [w3305]
              tunnel: [w3304] -> w3213
              tunnel: [w3303] -> w3211
              tunnel: w3215 -> [w3334]
              tunnel: [w3333] -> w3214
              tunnel: w3213 -> [w3333]
              tunnel: [w3332] -> w3212
              tunnel: w3211 -> [w3332]
              tunnel: w3214 -> [w3340]
              tunnel: w3212 -> [w3339]
              frame #0 {
                n2400 = local write "Puase for Loading"(TRUE ("Puase for Loading")) -> ()
              }
              frame #1 {
                n2401 = call "load config"() -> ("selected path"=w3256:path, "cancelled"=w3255:bool)  [unwired: 12 in, 2 out]
                n2402 = case shown="False" w3255 {
                  tunnel: w3257 -> [w3259 _]
                  tunnel: w3256 -> [w3260 _]
                  tunnel: [w3258 _] -> w3253
                  frame False {
                    n2403 = local write "config file"(w3260) -> ()
                    n2404 = call "Read and Write Controls to Automatic Config File.vi"("Action"=RWC_Actions."Read", "Control References"=w3259, "filepath"=w3260) -> ("error out"=w3258:errorcluster)  [unwired: 8 in]
                  }
                  frame True {
                  }
                }
              }
              frame #2 {
                n2405 = control-ref of="PhaseA Experiment Option"() -> (w3273:refnum<vi>)
                n2406 = control-ref of="PhaseG Experiment Option"() -> (w3272:refnum<vi>)
                n2407 = control-ref of="PhaseB Experiment Option"() -> (w3271:refnum<vi>)
                n2408 = control-ref of="PhaseH Experiment Option"() -> (w3270:refnum<vi>)
                n2409 = control-ref of="PhaseI Experiment Option"() -> (w3269:refnum<vi>)
                n2410 = control-ref of="PhaseC Experiment Option"() -> (w3268:refnum<vi>)
                n2411 = control-ref of="PhaseD Experiment Option"() -> (w3267:refnum<vi>)
                n2412 = control-ref of="PhaseE Experiment Option"() -> (w3266:refnum<vi>)
                n2413 = control-ref of="PhaseF Experiment Option"() -> (w3265:refnum<vi>)
                n2414 = control-ref of="PhaseL Experiment Option"() -> (w3264:refnum<vi>)
                n2415 = control-ref of="PhaseK Experiment Option"() -> (w3263:refnum<vi>)
                n2416 = control-ref of="PhaseJ Experiment Option"() -> (w3262:refnum<vi>)
                n2417 = control-ref of="How Many Experimental Phases?"() -> (w3298:refnum<vi>)
                n2418 = property class="DigNum (strict)"(reference=w3298) -> (reference out=w3300:refnum<vi>, "Value"=w3299:i32)  [unwired: 1 in, 1 out]
                n2419 = property class="CmbBox"(reference=w3273) -> (reference out=w3297:refnum<vi>, "Value"=w3296:string)  [unwired: 1 in, 1 out]
                n2420 = property class="CmbBox"(reference=w3272) -> (reference out=w3295:refnum<vi>, "Value"=w3294:string)  [unwired: 1 in, 1 out]
                n2421 = property class="CmbBox"(reference=w3271) -> (reference out=w3293:refnum<vi>, "Value"=w3292:string)  [unwired: 1 in, 1 out]
                n2422 = property class="CmbBox"(reference=w3270) -> (reference out=w3291:refnum<vi>, "Value"=w3290:string)  [unwired: 1 in, 1 out]
                n2423 = property class="CmbBox"(reference=w3269) -> (reference out=w3289:refnum<vi>, "Value"=w3288:string)  [unwired: 1 in, 1 out]
                n2424 = property class="CmbBox"(reference=w3268) -> (reference out=w3287:refnum<vi>, "Value"=w3286:string)  [unwired: 1 in, 1 out]
                n2425 = property class="CmbBox"(reference=w3267) -> (reference out=w3285:refnum<vi>, "Value"=w3284:string)  [unwired: 1 in, 1 out]
                n2426 = property class="CmbBox"(reference=w3266) -> (reference out=w3283:refnum<vi>, "Value"=w3282:string)  [unwired: 1 in, 1 out]
                n2427 = property class="CmbBox"(reference=w3265) -> (reference out=w3281:refnum<vi>, "Value"=w3280:string)  [unwired: 1 in, 1 out]
                n2428 = property class="CmbBox"(reference=w3264) -> (reference out=w3279:refnum<vi>, "Value"=w3278:string)  [unwired: 1 in, 1 out]
                n2429 = property class="CmbBox"(reference=w3263) -> (reference out=w3277:refnum<vi>, "Value"=w3276:string)  [unwired: 1 in, 1 out]
                n2430 = property class="CmbBox"(reference=w3262) -> (reference out=w3275:refnum<vi>, "Value"=w3274:string)  [unwired: 1 in, 1 out]
              }
              frame #3 {
                n2431 = property class="CmbBox"(reference=w3328, "Val(Sgnl)"=w3327) -> ()  [unwired: 1 in, 2 out]
                n2432 = property class="CmbBox"(reference=w3326, "Val(Sgnl)"=w3325) -> ()  [unwired: 1 in, 2 out]
                n2433 = property class="CmbBox"(reference=w3324, "Val(Sgnl)"=w3323) -> ()  [unwired: 1 in, 2 out]
                n2434 = property class="CmbBox"(reference=w3322, "Val(Sgnl)"=w3321) -> ()  [unwired: 1 in, 2 out]
                n2435 = property class="CmbBox"(reference=w3320, "Val(Sgnl)"=w3319) -> ()  [unwired: 1 in, 2 out]
                n2436 = property class="CmbBox"(reference=w3318, "Val(Sgnl)"=w3317) -> ()  [unwired: 1 in, 2 out]
                n2437 = property class="CmbBox"(reference=w3316, "Val(Sgnl)"=w3315) -> ()  [unwired: 1 in, 2 out]
                n2438 = property class="CmbBox"(reference=w3314, "Val(Sgnl)"=w3313) -> ()  [unwired: 1 in, 2 out]
                n2439 = property class="CmbBox"(reference=w3312, "Val(Sgnl)"=w3311) -> ()  [unwired: 1 in, 2 out]
                n2440 = property class="CmbBox"(reference=w3310, "Val(Sgnl)"=w3309) -> ()  [unwired: 1 in, 2 out]
                n2441 = property class="CmbBox"(reference=w3308, "Val(Sgnl)"=w3307) -> ()  [unwired: 1 in, 2 out]
                n2442 = property class="CmbBox"(reference=w3306, "Val(Sgnl)"=w3305) -> ()  [unwired: 1 in, 2 out]
                n2443 = local write "Puase for Loading"(FALSE ("Puase for Loading")) -> ()
                n2444 = property class="Bool (strict)"(reference=w3331, "Value"=FALSE) -> ()  [unwired: 1 in, 2 out]
              }
              frame #4 {
                n2445 = local read "Waveform Simulation Jump Filter (Hz)"() -> (w3336:dbl)
                n2446 = local read "Waveform Simulation sampling rate (Hz)"() -> (w3335:i32)
                n2447 = local read "How Many Experimental Phases?"() -> (w3337:i32)
                n2448 = call "clearOrCalcAllPhaseWaveforms_v02.vi"("How Many Experimental Phases?"=w3337, "Clear Waveform?"=FALSE, "Waveform Simulation Jump Filter (Hz)"=w3336, "Waveform Simulation sampling rate (Hz)"=w3335, "ExperimentOptionsCluster"=w3334) -> ()  [unwired: 6 in, 1 out]
              }
              frame #5 {
                n2449 = property class="DigNum (strict)"(reference=w3340, "Val(Sgnl)"=w3339) -> ()  [unwired: 1 in, 2 out]
                n2450 = One Button Dialog(message="Finished Loading" ("string"), button name ("OK")="click to resume") -> ()  [unwired: 1 out]
              }
            }
          }
        }
      }
    }
  }
  "config file" <- "protocol config"
  "Phase A" <- w340
  "Phase A Exp Option" <- w339
  "Phase B" <- w340
  "Phase B Exp Option" <- w339
  "Phase C" <- w340
  "Phase C Exp Option" <- w339
  "Phase D" <- w340
  "Phase D Exp Option" <- w339
  "Phase E" <- w340
  "Phase E Exp Option" <- w339
  "Phase F" <- w340
  "Phase F Exp Option" <- w339
  "Phase G" <- w340
  "Phase G Exp Option" <- w339
  "Phase H" <- w340
  "Phase H Exp Option" <- w339
  "Phase I" <- w340
  "Phase I Exp Option" <- w339
  "Phase J" <- w340
  "Phase J Exp Option" <- w339
  "Phase K" <- w340
  "Phase K Exp Option" <- w339
  "Phase L" <- w340
  "Phase L Exp Option" <- w339
  "Phase A Done" <- w338
  "Phase B Done" <- w338
  "Phase C Done" <- w338
  "Phase D Done" <- w338
  "Phase E Done" <- w338
  "Phase F Done" <- w338
  "Phase G Done" <- w338
  "Phase H Done" <- w338
  "Phase I Done" <- w338
  "Phase J Done" <- w338
  "Phase K Done" <- w338
  "Phase L Done" <- w338
